vi "FlexMag - 23-03-2023.vi"() -> ()   [LabVIEW 2018] (continued)
                  n22734 = case shown="False" w26543 {
                    frame False {
                      n22735 = local read "process file list"() -> (w26547:string)
                      n22736 = Match Pattern(string=w26547, regular expression="1-)") -> (after substring=w26544:string)  [unwired: 1 in, 3 out]
                      n22737 = Equal?(x="", y=w26544) -> (x = y?=w26546:bool)
                      n22738 = case shown="False" w26546 {
                        frame False {
                          # "process done"
                          n22739 = flat-sequence {
                            frame #0 {
                              n22740 = local write "coating process done"(TRUE ("coating process done")) -> ()
                              n22741 = local write "Buzzer DO"(TRUE ("Buzzer DO")) -> ()
                              n22742 = local write "coating start"(FALSE ("coating start")) -> ()
                              n22743 = local write "Stop auto LN2"(TRUE ("Stop auto LN2")) -> ()
                              n22744 = local write "System Status"("DEPOSITION DONE" ("Warning Message")) -> ()
                              n22745 = Wait (ms)(milliseconds to wait=u32 3000) -> ()  [unwired: 1 out]
                            }
                            frame #1 {
                            }
                            frame #2 {
                              n22746 = Wait (ms)(milliseconds to wait=u32 1000) -> ()  [unwired: 1 out]
                              n22747 = local write "Buzzer DO"(FALSE ("Buzzer DO")) -> ()
                            }
                          }
                        }
                        frame True {
                          # "wrong file"
                          n22748 = flat-sequence {
                            frame #0 {
                              n22749 = local write "Buzzer DO"(TRUE ("Buzzer DO")) -> ()
                              n22750 = local write "coating process done"(TRUE ("coating process done")) -> ()
                              n22751 = Wait (ms)(milliseconds to wait=u32 3000) -> ()  [unwired: 1 out]
                              n22752 = local write "coating start"(FALSE ("coating start")) -> ()
                              n22753 = local write "Warning Message"("Please Enter a proper Process File !" ("Warning Message")) -> ()
                            }
                            frame #1 {
                            }
                            frame #2 {
                              n22754 = Wait (ms)(milliseconds to wait=u32 1000) -> ()  [unwired: 1 out]
                              n22755 = local write "Buzzer DO"(FALSE ("Buzzer DO")) -> ()
                            }
                          }
                        }
                      }
                    }
                    frame True {
                    }
                  }
                }
              }
            }
          }
        }
        n22756 = local write "coating process done"(FALSE ("coating process done")) -> ()
      }
    }
  }
  n22757 = while {
    stop <- FALSE stop-if-true
    n22758 = Wait Until Next ms Multiple(millisecond multiple=u32 300 ("milliseconds to wait")) -> ()  [unwired: 1 out]
    n22759 = case shown="True" "dcps check active" {
      frame False {
      }
      frame True {
        n22760 = local read "Dcps_is_on"() -> (w26575:bool)
        n22761 = feedback #343() -> (w26574:bool)  [unwired: 1 in]
        n22762 = case shown="True" w26575 {
          tunnel: w26574 -> [_ w26578]
          tunnel: [TRUE ("coating start") w26577] -> w26573
          frame False {
          }
          frame True {
            n22763 = local read "Actual DC Power : 2"() -> (w26580:dbl)
            n22764 = local read "Set DC Power auto"() -> (w26583:dbl)
            n22765 = Add(x="power difference", y=w26580) -> (x+y=w26585:dbl)
            n22766 = Subtract(x=w26580, y="power difference") -> (x-y=w26584:dbl)
            n22767 = In Range and Coerce(upper limit=w26585, x=w26583, lower limit=w26584) -> (In Range?=w26582:bool)  [unwired: 1 out]
            n22768 = Not(x=w26582) -> (.not. x?=w26581:bool)
            n22769 = case shown="True" w26581 {
              tunnel: w26578 -> [_ w26587]
              tunnel: [TRUE ("coating process done") FALSE ("coating start")] -> w26577
              frame False {
              }
              frame True {
                n22770 = call "Elapsed Time192"("Reset"=w26587) -> ("Elapsed Time (s)"=w26590:dbl)  [unwired: 11 in, 7 out]
                n22771 = Greater Or Equal?(x=w26590, y="dcps check(sec)") -> (x >= y?=w26589:bool)
                n22772 = case shown="True" w26589 {
                  frame False {
                  }
                  frame True {
                    n22773 = local read "coating start"() -> (w26594:bool)
                    n22774 = case shown="True" w26594 {
                      frame False {
                      }
                      frame True {
                        n22775 = local write "coating error"(TRUE ("coating error")) -> ()
                      }
                    }
                    n22776 = local write "Dc_auto_off"(TRUE ("Dc_auto_off")) -> ()
                    n22777 = local write "Warning Message"("No Actual  DC Power !" ("Warning Message")) -> ()
                  }
                }
              }
            }
          }
        }
        n22778 = feedback-in #343(w26573) -> ()
      }
    }
    n22779 = feedback #344() -> (w26568:bool)  [unwired: 1 in]
    n22780 = feedback #345() -> (w26569:bool)  [unwired: 1 in]
    n22781 = case shown="True" "coating error" {
      tunnel: [TRUE FALSE] -> w26567
      tunnel: w26568 -> [_ w26604]
      frame False {
      }
      frame True {
        n22782 = call "Elapsed Time156"("Auto Reset"=w26604) -> ("Elapsed Time (s)"=w26599:dbl)  [unwired: 11 in, 7 out]
        n22783 = In Range and Coerce(upper limit=7.0, x=w26599, lower limit=2.0) -> (In Range?=w26602:bool)  [unwired: 1 out]
        n22784 = In Range and Coerce(upper limit=1.5, x=w26599, lower limit=0.0) -> (In Range?=w26603:bool)  [unwired: 1 out]
        n22785 = In Range and Coerce(upper limit=10.0, x=w26599, lower limit=9.0) -> (In Range?=w26598:bool)  [unwired: 1 out]
        n22786 = case shown="True" w26603 {
          frame False {
          }
          frame True {
            w26622 = FALSE ("forward roll")
            w26623 = FALSE ("forward roll")
            n22787 = local write "coating process done"(TRUE ("coating process done")) -> ()
            n22788 = local write "Buzzer DO"(TRUE ("coating process done")) -> ()
            n22789 = local write "coating start"(FALSE ("coating start")) -> ()
            n22790 = local write "System Status"("COATING PROCESS CANCELLED !" ("System Status")) -> ()
            n22791 = local write "MFC_Ar_Set_value"(0.0 ("MFC_Ar_Set_value")) -> ()
            n22792 = local write "forward roll"(w26623) -> ()
            n22793 = local write "back roll"(w26623) -> ()
            n22794 = local write "CH1_Motor DO"(w26622) -> ()
            n22795 = local write "CH2_Motor DO"(w26622) -> ()
            n22796 = local write "CH3_Motor DO"(w26622) -> ()
            n22797 = local write "CH4_Motor DO"(w26622) -> ()
          }
        }
        n22798 = case shown="True" w26602 {
          frame False {
          }
          frame True {
            w26618 = TRUE ("Dc_auto_off")
            n22799 = local write "coating start"(FALSE ("coating start")) -> ()
            n22800 = local write "Dc_auto_off"(w26618) -> ()
            n22801 = local write "RF_auto_off"(w26618) -> ()
            n22802 = local write "MWPS1 auto close"(w26618) -> ()
            n22803 = local write "MWPS2 auto close"(w26618) -> ()
            n22804 = local write "MFC_Ar_Set"(TRUE ("MFC_Ar_Set")) -> ()
            n22805 = local write "Buzzer DO"(FALSE ("Buzzer DO")) -> ()
          }
        }
        n22806 = case shown="True" w26598 {
          frame False {
          }
          frame True {
            n22807 = local write "MFC_Ar_Set"(FALSE ("MFC_Ar_Set")) -> ()
            n22808 = local write "System Status"("SEMI-AUTOMATIC MODE" ("System Status")) -> ()
            n22809 = local write "coating error"(FALSE ("stop coating")) -> ()
          }
        }
        n22810 = local read "cassette position selection"() -> (w26597:u16)
        n22811 = case shown="4" w26597 {
          frame 0, Default {
          }
          frame 1 {
            n22812 = local write "pcgv1 auto open"(TRUE ("pcgv1 auto open")) -> ()
          }
          frame 2 {
            n22813 = local write "pcgv2 auto open"(TRUE ("pcgv2 auto open")) -> ()
          }
          frame 3 {
            n22814 = local write "pcgv3 auto open"(TRUE ("Dc_auto_off")) -> ()
          }
          frame 4 {
            n22815 = local write "pcgv4 auto open"(TRUE ("Dc_auto_off")) -> ()
          }
        }
      }
    }
    n22816 = feedback-in #344(w26567) -> ()
    n22817 = case shown="True" "stop coating" {
      tunnel: [TRUE FALSE] -> w26571
      tunnel: w26569 -> [_ w26636]
      frame False {
      }
      frame True {
        n22818 = call "Elapsed Time155"("Auto Reset"=w26636) -> ("Elapsed Time (s)"=w26631:dbl)  [unwired: 11 in, 7 out]
        n22819 = In Range and Coerce(upper limit=4.0, x=w26631, lower limit=2.0) -> (In Range?=w26634:bool)  [unwired: 1 out]
        n22820 = In Range and Coerce(upper limit=1.5, x=w26631, lower limit=0.0) -> (In Range?=w26635:bool)  [unwired: 1 out]
        n22821 = In Range and Coerce(upper limit=10.0, x=w26631, lower limit=7.0) -> (In Range?=w26630:bool)  [unwired: 1 out]
        n22822 = case shown="True" w26635 {
          frame False {
          }
          frame True {
            w26654 = FALSE ("forward roll")
            w26655 = FALSE ("forward roll")
            w26656 = TRUE ("coating process done")
            n22823 = local write "Buzzer DO"(w26656) -> ()
            n22824 = local write "coating process done"(w26656) -> ()
            n22825 = local write "coating start"(FALSE ("coating start")) -> ()
            n22826 = local write "System Status"("COATING PROCESS CANCELLED !" ("System Status")) -> ()
            n22827 = local write "MFC_Ar_Set_value"(0.0 ("MFC_Ar_Set_value")) -> ()
            n22828 = local write "forward roll"(w26655) -> ()
            n22829 = local write "back roll"(w26655) -> ()
            n22830 = local write "CH1_Motor DO"(w26654) -> ()
            n22831 = local write "CH2_Motor DO"(w26654) -> ()
            n22832 = local write "CH3_Motor DO"(w26654) -> ()
            n22833 = local write "CH4_Motor DO"(w26654) -> ()
          }
        }
        n22834 = case shown="True" w26634 {
          frame False {
          }
          frame True {
            w26650 = TRUE ("Dc_auto_off")
            n22835 = local write "coating start"(FALSE ("coating start")) -> ()
            n22836 = local write "Dc_auto_off"(w26650) -> ()
            n22837 = local write "RF_auto_off"(w26650) -> ()
            n22838 = local write "MWPS1 auto close"(w26650) -> ()
            n22839 = local write "MWPS2 auto close"(w26650) -> ()
            n22840 = local write "MFC_Ar_Set"(TRUE ("MFC_Ar_Set")) -> ()
            n22841 = local write "Buzzer DO"(FALSE ("Buzzer DO")) -> ()
          }
        }
        n22842 = case shown="True" w26630 {
          frame False {
          }
          frame True {
            n22843 = local write "MFC_Ar_Set"(FALSE ("MFC_Ar_Set")) -> ()
            n22844 = local write "stop coating"(FALSE ("stop coating")) -> ()
            n22845 = local write "System Status"("SEMI-AUTOMATIC MODE" ("System Status")) -> ()
          }
        }
        n22846 = local read "cassette position selection"() -> (w26629:u16)
        n22847 = case shown="4" w26629 {
          frame 0, Default {
          }
          frame 1 {
            n22848 = local write "pcgv1 auto open"(TRUE ("pcgv1 auto open")) -> ()
          }
          frame 2 {
            n22849 = local write "pcgv2 auto open"(TRUE ("pcgv2 auto open")) -> ()
          }
          frame 3 {
            n22850 = local write "pcgv3 auto open"(TRUE ("Dc_auto_off")) -> ()
          }
          frame 4 {
            n22851 = local write "pcgv4 auto open"(TRUE ("Dc_auto_off")) -> ()
          }
        }
      }
    }
    n22852 = feedback-in #345(w26571) -> ()
  }
  n22853 = while {
    stop <- FALSE stop-if-true
    n22854 = Wait Until Next ms Multiple(millisecond multiple=u32 300) -> ()  [unwired: 1 out]
    n22855 = case shown="True" "load process file" {
      frame False {
      }
      frame True {
        n22856 = stacked-sequence {
          seq-local: [w26670 _ _] -> [_ w26677 _]
          frame #0 {
            n22857 = call "File Dialog"("start path"=path "D:/VK-1701 System Files/Process Files") -> ("selected path"=w26672:path, "cancelled"=w26669:bool, "error out"=→"error out":errorcluster)  [unwired: 11 in, 1 out]
            n22858 = case shown="False" w26669 {
              tunnel: w26672 -> [w26675 _]
              tunnel: [w26674 string[][] [] ("all rows")] -> w26670
              frame False {
                n22859 = call-poly <vilib>:"Read Delimited Spreadsheet.vi"("file path (dialog if empty)"=w26675) -> ("all rows"=w26674:string[][])  [unwired: 9 in, 5 out]
              }
              frame True {
              }
            }
            "process counter" <- 0.0 ("Numeric")
            "process file list" <- "" ("process file list")
          }
          frame #1 {
            n22860 = while {
              tunnel: w26677 -> [w26683]
              i -> [w26682]
              stop <- w26679 stop-if-true
              n22861 = Index Array(array=w26683, index (row)=w26682, index (col)=0 ("disabled index (col)")) -> (element=w26678:string)
              n22862 = Equal?(x=w26678, y="") -> (x = y?=w26679:bool)
              n22863 = case shown="False" w26679 {
                tunnel: w26678 -> [w26684 _]
                frame False {
                  n22864 = local read "process file list"() -> (w26686:string)
                  n22865 = Concatenate Strings(w26686, "\r\n", w26684) -> (w26687:string)
                  n22866 = local write "process file list"(w26687) -> ()
                }
                frame True {
                }
              }
            }
          }
          frame #2 {
            n22867 = local read "process file list"() -> (w26690:string)
            n22868 = Match Pattern(string=w26690, regular expression="\r\n") -> (after substring=w26688:string)  [unwired: 1 in, 3 out]
            n22869 = local write "process file list"(w26688) -> ()
          }
        }
      }
    }
    n22870 = case shown="True" "creat recipe file" {
      frame False {
      }
      frame True {
        n22871 = call "FlexMag recipe file.vi"() -> ()  [unwired: 2 in]
      }
    }
    n22872 = case shown="True" "Change Rolling Direction" {
      frame False {
      }
      frame True {
        n22873 = local read "dep. for?"() -> (w26666:bool)
        n22874 = Not(x=w26666) -> (.not. x?=w26665:bool)
        n22875 = local write "dep. for?"(w26665) -> ()
        n22876 = local write "rolling direction gui"(w26665) -> ()
      }
    }
    n22877 = case shown="True" "creat process file" {
      frame False {
      }
      frame True {
        n22878 = call "FlexMag process file.vi"() -> ()  [unwired: 12 in]
      }
    }
  }
  n22879 = while {
    stop <- FALSE stop-if-true
    n22880 = Wait Until Next ms Multiple(millisecond multiple=u32 300) -> ()  [unwired: 1 out]
    n22881 = case shown="True" "CH1 LN2" {
      frame False {
      }
      frame True {
        n22882 = stacked-sequence {
          frame #0 {
            n22883 = local write "CH1_LN2_DO"(TRUE ("CH1_LN2_DO")) -> ()
            n22884 = Wait (ms)(milliseconds to wait=u32 100) -> ()  [unwired: 1 out]
          }
          frame #1 {
            n22885 = while {
              stop <- w26697 stop-if-true
              n22886 = stacked-sequence {
                frame #0 {
                  n22887 = while {
                    stop <- w26702 stop-if-true
                    n22888 = local read "ln2 ch1 top aim"() -> (w26704:dbl)
                    n22889 = local read "CH1_LN2_TK_t"() -> (w26705:u16)
                    n22890 = local read "CH1 LN2"() -> (w26703:bool)
                    n22891 = Greater Or Equal?(x=w26705, y=w26704) -> (x >= y?=w26701:bool)
                    n22892 = Not(x=w26703) -> (.not. x?=w26700:bool)
                    n22893 = Or(x=w26701, y=w26700) -> (x .or. y?=w26702:bool)
                    n22894 = Wait Until Next ms Multiple(millisecond multiple=u32 300) -> ()  [unwired: 1 out]
                  }
                }
                frame #1 {
                  n22895 = local write "CH1_LN2_DO"(FALSE ("CH1_LN2_DO")) -> ()
                  n22896 = Wait (ms)(milliseconds to wait=u32 100) -> ()  [unwired: 1 out]
                }
                frame #2 {
                  n22897 = while {
                    stop <- w26711 stop-if-true
                    n22898 = local read "ln2 ch1 bottom drop"() -> (w26713:dbl)
                    n22899 = local read "CH1_LN2_TK_b"() -> (w26714:u16)
                    n22900 = local read "CH1 LN2"() -> (w26712:bool)
                    n22901 = Less Or Equal?(x=w26714, y=w26713) -> (x <= y?=w26710:bool)
                    n22902 = Not(x=w26712) -> (.not. x?=w26709:bool)
                    n22903 = Or(x=w26710, y=w26709) -> (x .or. y?=w26711:bool)
                    n22904 = Wait Until Next ms Multiple(millisecond multiple=u32 300) -> ()  [unwired: 1 out]
                  }
                }
                frame #3 {
                  n22905 = local write "CH1_LN2_DO"(TRUE ("CH1_LN2_DO")) -> ()
                  n22906 = Wait (ms)(milliseconds to wait=u32 500) -> ()  [unwired: 1 out]
                }
                frame #4 {
                  n22907 = disable-structure shown="Disabled" {
                    frame Disabled {
                      n22908 = while {
                        stop <- w26721 stop-if-true
                        n22909 = local read "CH1_LN2_TK_t"() -> (w26723:u16)
                        n22910 = local read "ln2 dropdown"() -> (w26717:dbl)
                        n22911 = local read "CH1 LN2"() -> (w26722:bool)
                        n22912 = Less Or Equal?(x=w26723, y=w26717) -> (x <= y?=w26720:bool)
                        n22913 = Not(x=w26722) -> (.not. x?=w26719:bool)
                        n22914 = Or(x=w26720, y=w26719) -> (x .or. y?=w26721:bool)
                        n22915 = Wait Until Next ms Multiple(millisecond multiple=u32 300) -> ()  [unwired: 1 out]
                      }
                    }
                    frame Enabled {
                    }
                  }
                }
              }
              n22916 = Wait Until Next ms Multiple(millisecond multiple=u32 300) -> ()  [unwired: 1 out]
              n22917 = local read "CH1 LN2"() -> (w26698:bool)
              n22918 = Not(x=w26698) -> (.not. x?=w26697:bool)
            }
          }
          frame #2 {
            n22919 = local write "CH1_LN2_DO"(FALSE ("CH1_LN2_DO")) -> ()
            n22920 = Wait (ms)(milliseconds to wait=u32 100) -> ()  [unwired: 1 out]
          }
        }
      }
    }
  }
  n22921 = while {
    stop <- FALSE stop-if-true
    n22922 = Wait Until Next ms Multiple(millisecond multiple=u32 300) -> ()  [unwired: 1 out]
    n22923 = case shown="True" "CH2 LN2" {
      frame False {
      }
      frame True {
        n22924 = stacked-sequence {
          frame #0 {
            n22925 = local write "CH2_LN2_DO"(TRUE ("CH1_LN2_DO")) -> ()
            n22926 = Wait (ms)(milliseconds to wait=u32 100) -> ()  [unwired: 1 out]
          }
          frame #1 {
            n22927 = while {
              stop <- w26732 stop-if-true
              n22928 = stacked-sequence {
                frame #0 {
                  n22929 = while {
                    stop <- w26737 stop-if-true
                    n22930 = local read "ln2 ch2 top aim"() -> (w26739:dbl)
                    n22931 = local read "CH2_LN2_TK_t"() -> (w26740:u16)
                    n22932 = local read "CH2 LN2"() -> (w26738:bool)
                    n22933 = Greater Or Equal?(x=w26740, y=w26739) -> (x >= y?=w26736:bool)
                    n22934 = Not(x=w26738) -> (.not. x?=w26735:bool)
                    n22935 = Or(x=w26736, y=w26735) -> (x .or. y?=w26737:bool)
                    n22936 = Wait Until Next ms Multiple(millisecond multiple=u32 300) -> ()  [unwired: 1 out]
                  }
                }
                frame #1 {
                  n22937 = local write "CH2_LN2_DO"(FALSE ("CH1_LN2_DO")) -> ()
                  n22938 = Wait (ms)(milliseconds to wait=u32 100) -> ()  [unwired: 1 out]
                }
                frame #2 {
                  n22939 = while {
                    stop <- w26746 stop-if-true
                    n22940 = local read "ln2 ch3 bottom drop"() -> (w26748:dbl)
                    n22941 = local read "CH2_LN2_TK_b"() -> (w26749:u16)
                    n22942 = local read "CH2 LN2"() -> (w26747:bool)
                    n22943 = Less Or Equal?(x=w26749, y=w26748) -> (x <= y?=w26745:bool)
                    n22944 = Not(x=w26747) -> (.not. x?=w26744:bool)
                    n22945 = Or(x=w26745, y=w26744) -> (x .or. y?=w26746:bool)
                    n22946 = Wait Until Next ms Multiple(millisecond multiple=u32 300) -> ()  [unwired: 1 out]
                  }
                }
                frame #3 {
                  n22947 = local write "CH2_LN2_DO"(TRUE) -> ()
                  n22948 = Wait (ms)(milliseconds to wait=u32 500) -> ()  [unwired: 1 out]
                }
                frame #4 {
                  n22949 = disable-structure shown="Disabled" {
                    frame Disabled {
                      n22950 = while {
                        stop <- w26756 stop-if-true
                        n22951 = local read "CH2_LN2_TK_t"() -> (w26758:u16)
                        n22952 = local read "ln2 dropdown"() -> (w26752:dbl)
                        n22953 = local read "CH2 LN2"() -> (w26757:bool)
                        n22954 = Less Or Equal?(x=w26758, y=w26752) -> (x <= y?=w26755:bool)
                        n22955 = Not(x=w26757) -> (.not. x?=w26754:bool)
                        n22956 = Or(x=w26755, y=w26754) -> (x .or. y?=w26756:bool)
                        n22957 = Wait Until Next ms Multiple(millisecond multiple=u32 300) -> ()  [unwired: 1 out]
                      }
                    }
                    frame Enabled {
                    }
                  }
                }
              }
              n22958 = Wait Until Next ms Multiple(millisecond multiple=u32 300) -> ()  [unwired: 1 out]
              n22959 = local read "CH2 LN2"() -> (w26733:bool)
              n22960 = Not(x=w26733) -> (.not. x?=w26732:bool)
            }
          }
          frame #2 {
            n22961 = local write "CH2_LN2_DO"(FALSE ("CH2_LN2_DO")) -> ()
            n22962 = Wait (ms)(milliseconds to wait=u32 100) -> ()  [unwired: 1 out]
          }
        }
      }
    }
  }
  n22963 = while {
    stop <- FALSE stop-if-true
    n22964 = Wait Until Next ms Multiple(millisecond multiple=u32 300) -> ()  [unwired: 1 out]
    n22965 = case shown="True" "CH3 LN2" {
      frame False {
      }
      frame True {
        n22966 = stacked-sequence {
          frame #0 {
            n22967 = local write "CH3_LN2_DO"(TRUE ("CH1_LN2_DO")) -> ()
            n22968 = Wait (ms)(milliseconds to wait=u32 100) -> ()  [unwired: 1 out]
          }
          frame #1 {
            n22969 = while {
              stop <- w26767 stop-if-true
              n22970 = stacked-sequence {
                frame #0 {
                  n22971 = while {
                    stop <- w26772 stop-if-true
                    n22972 = local read "ln2 ch3 top aim"() -> (w26774:dbl)
                    n22973 = local read "CH3_LN2_TK_t"() -> (w26775:u16)
                    n22974 = local read "CH3 LN2"() -> (w26773:bool)
                    n22975 = Greater Or Equal?(x=w26775, y=w26774) -> (x >= y?=w26771:bool)
                    n22976 = Not(x=w26773) -> (.not. x?=w26770:bool)
                    n22977 = Or(x=w26771, y=w26770) -> (x .or. y?=w26772:bool)
                    n22978 = Wait Until Next ms Multiple(millisecond multiple=u32 300) -> ()  [unwired: 1 out]
                  }
                }
                frame #1 {
                  n22979 = local write "CH3_LN2_DO"(FALSE ("CH1_LN2_DO")) -> ()
                  n22980 = Wait (ms)(milliseconds to wait=u32 100) -> ()  [unwired: 1 out]
                }
                frame #2 {
                  n22981 = while {
                    stop <- w26781 stop-if-true
                    n22982 = local read "ln2 ch3 bottom drop"() -> (w26783:dbl)
                    n22983 = local read "CH3_LN2_TK_b"() -> (w26784:u16)
                    n22984 = local read "CH3 LN2"() -> (w26782:bool)
                    n22985 = Less Or Equal?(x=w26784, y=w26783) -> (x <= y?=w26780:bool)
                    n22986 = Not(x=w26782) -> (.not. x?=w26779:bool)
                    n22987 = Or(x=w26780, y=w26779) -> (x .or. y?=w26781:bool)
                    n22988 = Wait Until Next ms Multiple(millisecond multiple=u32 300) -> ()  [unwired: 1 out]
                  }
                }
                frame #3 {
                  n22989 = local write "CH3_LN2_DO"(TRUE) -> ()
                  n22990 = Wait (ms)(milliseconds to wait=u32 500) -> ()  [unwired: 1 out]
                }
                frame #4 {
                  n22991 = disable-structure shown="Disabled" {
                    frame Disabled {
                      n22992 = while {
                        stop <- w26791 stop-if-true
                        n22993 = local read "CH3_LN2_TK_t"() -> (w26793:u16)
                        n22994 = local read "ln2 dropdown"() -> (w26787:dbl)
                        n22995 = local read "CH3 LN2"() -> (w26792:bool)
                        n22996 = Less Or Equal?(x=w26793, y=w26787) -> (x <= y?=w26790:bool)
                        n22997 = Not(x=w26792) -> (.not. x?=w26789:bool)
                        n22998 = Or(x=w26790, y=w26789) -> (x .or. y?=w26791:bool)
                        n22999 = Wait Until Next ms Multiple(millisecond multiple=u32 300) -> ()  [unwired: 1 out]
                      }
                    }
                    frame Enabled {
                    }
                  }
                }
              }
              n23000 = Wait Until Next ms Multiple(millisecond multiple=u32 300) -> ()  [unwired: 1 out]
              n23001 = local read "CH3 LN2"() -> (w26768:bool)
              n23002 = Not(x=w26768) -> (.not. x?=w26767:bool)
            }
          }
          frame #2 {
            n23003 = local write "CH3_LN2_DO"(FALSE ("CH3_LN2_DO")) -> ()
            n23004 = Wait (ms)(milliseconds to wait=u32 100) -> ()  [unwired: 1 out]
          }
        }
      }
    }
  }
  n23005 = while {
    stop <- FALSE stop-if-true
    n23006 = Wait Until Next ms Multiple(millisecond multiple=u32 300) -> ()  [unwired: 1 out]
    n23007 = case shown="True" "CH4 LN2" {
      frame False {
      }
      frame True {
        n23008 = stacked-sequence {
          frame #0 {
            n23009 = local write "CH4_LN2_DO"(TRUE ("CH1_LN2_DO")) -> ()
            n23010 = Wait (ms)(milliseconds to wait=u32 100) -> ()  [unwired: 1 out]
          }
          frame #1 {
            n23011 = while {
              stop <- w26802 stop-if-true
              n23012 = stacked-sequence {
                frame #0 {
                  n23013 = while {
                    stop <- w26807 stop-if-true
                    n23014 = local read "ln2 ch4 top aim"() -> (w26809:dbl)
                    n23015 = local read "CH4_LN2_TK_t"() -> (w26810:u16)
                    n23016 = local read "CH4 LN2"() -> (w26808:bool)
                    n23017 = Greater Or Equal?(x=w26810, y=w26809) -> (x >= y?=w26806:bool)
                    n23018 = Not(x=w26808) -> (.not. x?=w26805:bool)
                    n23019 = Or(x=w26806, y=w26805) -> (x .or. y?=w26807:bool)
                    n23020 = Wait Until Next ms Multiple(millisecond multiple=u32 300) -> ()  [unwired: 1 out]
                  }
                }
                frame #1 {
                  n23021 = local write "CH4_LN2_DO"(FALSE ("CH1_LN2_DO")) -> ()
                  n23022 = Wait (ms)(milliseconds to wait=u32 100) -> ()  [unwired: 1 out]
                }
                frame #2 {
                  n23023 = while {
                    stop <- w26816 stop-if-true
                    n23024 = local read "ln2 ch4 bottom drop"() -> (w26818:dbl)
                    n23025 = local read "CH4_LN2_TK_b"() -> (w26819:u16)
                    n23026 = local read "CH4 LN2"() -> (w26817:bool)
                    n23027 = Less Or Equal?(x=w26819, y=w26818) -> (x <= y?=w26815:bool)
                    n23028 = Not(x=w26817) -> (.not. x?=w26814:bool)
                    n23029 = Or(x=w26815, y=w26814) -> (x .or. y?=w26816:bool)
                    n23030 = Wait Until Next ms Multiple(millisecond multiple=u32 300) -> ()  [unwired: 1 out]
                  }
                }
                frame #3 {
                  n23031 = local write "CH4_LN2_DO"(TRUE ("CH4_LN2_DO")) -> ()
                  n23032 = Wait (ms)(milliseconds to wait=u32 500) -> ()  [unwired: 1 out]
                }
                frame #4 {
                  n23033 = disable-structure shown="Disabled" {
                    frame Disabled {
                      n23034 = while {
                        stop <- w26826 stop-if-true
                        n23035 = local read "CH4_LN2_TK_t"() -> (w26828:u16)
                        n23036 = local read "ln2 dropdown"() -> (w26822:dbl)
                        n23037 = local read "CH4 LN2"() -> (w26827:bool)
                        n23038 = Less Or Equal?(x=w26828, y=w26822) -> (x <= y?=w26825:bool)
                        n23039 = Not(x=w26827) -> (.not. x?=w26824:bool)
                        n23040 = Or(x=w26825, y=w26824) -> (x .or. y?=w26826:bool)
                        n23041 = Wait Until Next ms Multiple(millisecond multiple=u32 300) -> ()  [unwired: 1 out]
                      }
                    }
                    frame Enabled {
                    }
                  }
                }
              }
              n23042 = Wait Until Next ms Multiple(millisecond multiple=u32 300) -> ()  [unwired: 1 out]
              n23043 = local read "CH4 LN2"() -> (w26803:bool)
              n23044 = Not(x=w26803) -> (.not. x?=w26802:bool)
            }
          }
          frame #2 {
            n23045 = local write "CH4_LN2_DO"(FALSE ("CH4_LN2_DO")) -> ()
            n23046 = Wait (ms)(milliseconds to wait=u32 100) -> ()  [unwired: 1 out]
          }
        }
      }
    }
  }
  n23047 = while {
    stop <- FALSE stop-if-true
    n23048 = Wait Until Next ms Multiple(millisecond multiple=u32 300) -> ()  [unwired: 1 out]
    n23049 = case shown="True" "Stop auto LN2" {
      frame False {
      }
      frame True {
        w26836 = FALSE ("CH1 LN2")
        w26837 = FALSE ("CH1 LN2")
        n23050 = local write "CH1_LN2_DO"(w26836) -> ()
        n23051 = local write "CH2_LN2_DO"(w26836) -> ()
        n23052 = local write "CH3_LN2_DO"(w26836) -> ()
        n23053 = local write "CH4_LN2_DO"(w26836) -> ()
        n23054 = local write "Stop auto LN2"(FALSE ("CH1 LN2")) -> ()
        n23055 = local write "CH1 LN2"(w26837) -> ()
        n23056 = local write "CH2 LN2"(w26837) -> ()
        n23057 = local write "CH3 LN2"(w26837) -> ()
        n23058 = local write "CH4 LN2"(w26837) -> ()
        n23059 = Wait (ms)(milliseconds to wait=u32 100) -> ()  [unwired: 1 out]
      }
    }
  }
  n23060 = while {
    stop <- FALSE stop-if-true
    n23061 = local read "CH1 LN2"() -> (w26842:bool)
    n23062 = local read "CH2 LN2"() -> (w26841:bool)
    n23063 = local read "CH3 LN2"() -> (w26840:bool)
    n23064 = local read "CH4 LN2"() -> (w26839:bool)
    n23065 = Wait Until Next ms Multiple(millisecond multiple=u32 1000) -> ()  [unwired: 1 out]
    n23066 = Compound Arithmetic op=OR(w26842, w26841, w26840, w26839) -> (w26843:bool)
    n23067 = case shown="True" w26843 {
      tunnel: [FALSE w26849] -> w26838
      frame False {
      }
      frame True {
        n23068 = local read "CH1_LN2_TK_b"() -> (w26863:u16)
        n23069 = local read "CH2_LN2_TK_b"() -> (w26856:u16)
        n23070 = local read "CH3_LN2_TK_b"() -> (w26858:u16)
        n23071 = local read "CH4_LN2_TK_b"() -> (w26859:u16)
        n23072 = local read "error level"() -> (w26862:dbl)
        n23073 = local read "error level"() -> (w26861:dbl)
        n23074 = local read "error level"() -> (w26857:dbl)
        n23075 = local read "error level"() -> (w26860:dbl)
        n23076 = Less Or Equal?(x=w26863, y=w26862) -> (x <= y?=w26855:bool)
        n23077 = Less Or Equal?(x=w26856, y=w26861) -> (x <= y?=w26853:bool)
        n23078 = Less Or Equal?(x=w26858, y=w26857) -> (x <= y?=w26852:bool)
        n23079 = Less Or Equal?(x=w26859, y=w26860) -> (x <= y?=w26851:bool)
        n23080 = Compound Arithmetic op=AND(w26855, w26853, w26852, w26851) -> (w26850:bool)
        n23081 = feedback #346() -> (w26864:bool)  [unwired: 1 in]
        n23082 = case shown="True" w26850 {
          tunnel: [TRUE FALSE] -> w26854
          tunnel: w26864 -> [_ w26870]
          tunnel: [FALSE w26871] -> w26849
          frame False {
          }
          frame True {
            n23083 = call "Elapsed Time189"("Reset"=w26870) -> ("Elapsed Time (s)"=w26872:dbl)  [unwired: 11 in, 7 out]
            n23084 = Multiply(x=60.0, y="dewar error time(min)") -> (x*y=w26869:dbl)
            n23085 = Greater Or Equal?(x=w26872, y=w26869) -> (x >= y?=w26871:bool)
          }
        }
        n23086 = feedback-in #346(w26854) -> ()
      }
    }
    n23087 = case shown="True" w26838 {
      frame False {
      }
      frame True {
        n23088 = local write "Warning Message"("Dewar is empty !") -> ()
        n23089 = local write "Stop auto LN2"(TRUE ("CH1 LN2")) -> ()
      }
    }
  }
  n23090 = VISA Close(VISA resource name=w60, error in (no error)=w61) -> ()  [unwired: 1 out]
  n23091 = while {
    stop <- FALSE stop-if-true
    n23092 = Wait Until Next ms Multiple(millisecond multiple=u32 300) -> ()  [unwired: 1 out]
    n23093 = case shown="True" "load recipe from path" {
      frame False {
      }
      frame True {
        n23094 = stacked-sequence {
          frame #0 {
            n23095 = local read "path for loading recipe"() -> (w27046:path)
            n23096 = call-poly <vilib>:"Read Delimited Spreadsheet.vi"("file path (dialog if empty)"=w27046) -> ("all rows"=w27166:string[][])  [unwired: 9 in, 5 out]
            n23097 = Index Array(array=w27166, index (row) #1=0 ("index (row)"), index (col) #1=4 ("index (row)"), index (row) #2=1 ("index (row)"), index (col) #2=4 ("index (row)"), index (row) #3=4 ("index (row)"), index (col) #3=4 ("index (row)"), index (row) #4=5 ("index (row)"), index (col) #4=4 ("index (row)"), index (row) #5=8 ("index (row)"), index (col) #5=4 ("index (row)"), index (row) #6=9 ("index (row)"), index (col) #6=4 ("index (row)"), index (row) #7=10 ("index (row)"), index (col) #7=4 ("index (row)"), index (row) #8=13 ("index (row)"), index (col) #8=4 ("index (row)"), index (row) #9=14 ("index (row)"), index (col) #9=4 ("index (row)"), index (row) #10=17 ("index (row)"), index (col) #10=4 ("index (row)"), index (row) #11=18 ("index (row)"), index (col) #11=4 ("index (row)"), index (row) #12=21 ("index (row)"), index (col) #12=4 ("index (row)"), index (row) #13=28 ("index (row)"), index (col) #13=4 ("index (row)"), index (row) #14=29 ("index (row)"), index (col) #14=4 ("index (row)"), index (row) #15=30 ("index (row)"), index (col) #15=4 ("index (row)"), index (row) #16=31 ("index (row)"), index (col) #16=4 ("index (row)"), index (row) #17=32 ("index (row)"), index (col) #17=4 ("index (row)"), index (row) #18=33 ("index (row)"), index (col) #18=4 ("index (row)"), index (row) #19=34 ("index (row)"), index (col) #19=4 ("index (row)"), index (row) #20=35 ("index (row)"), index (col) #20=4 ("index (row)"), index (row) #21=36 ("index (row)"), index (col) #21=4 ("index (row)"), index (row) #22=37 ("index (row)"), index (col) #22=4 ("index (row)"), index (row) #23=38 ("index (row)"), index (col) #23=4 ("index (row)"), index (row) #24=39 ("index (row)"), index (col) #24=4 ("index (row)"), index (row) #25=40 ("index (row)"), index (col) #25=4 ("index (row)"), index (row) #26=41 ("index (row)"), index (col) #26=4 ("index (row)"), index (row) #27=42 ("index (row)"), index (col) #27=4 ("index (row)"), index (row) #28=43 ("index (row)"), index (col) #28=4 ("index (row)"), index (row) #29=44 ("index (row)"), index (col) #29=4 ("index (row)"), index (row) #30=45 ("index (row)"), index (col) #30=4 ("index (row)"), index (row) #31=46 ("index (row)"), index (col) #31=4 ("index (row)"), index (row) #32=47 ("index (row)"), index (col) #32=4 ("index (row)"), index (row) #33=50 ("index (row)"), index (col) #33=4 ("index (row)"), index (row) #34=51 ("index (row)"), index (col) #34=4 ("index (row)"), index (row) #35=52 ("index (row)"), index (col) #35=4 ("index (row)"), index (row) #36=53 ("index (row)"), index (col) #36=4 ("index (row)"), index (row) #37=54 ("index (row)"), index (col) #37=4 ("index (row)"), index (row) #38=55 ("index (row)"), index (col) #38=4 ("index (row)"), index (row) #39=56 ("index (row)"), index (col) #39=4 ("index (row)"), index (row) #40=57 ("index (row)"), index (col) #40=4 ("index (row)"), index (row) #41=58 ("index (row)"), index (col) #41=4 ("index (row)"), index (row) #42=59 ("index (row)"), index (col) #42=4 ("index (row)"), index (row) #43=60 ("index (row)"), index (col) #43=4 ("index (row)"), index (row) #44=61 ("index (row)"), index (col) #44=4 ("index (row)"), index (row) #45=62 ("index (row)"), index (col) #45=4 ("index (row)"), index (row) #46=63 ("index (row)"), index (col) #46=4 ("index (row)"), index (row) #47=64 ("index (row)"), index (col) #47=4 ("index (row)"), index (row) #48=65 ("index (row)"), index (col) #48=4 ("index (row)"), index (row) #49=66 ("index (row)"), index (col) #49=4 ("index (row)"), index (row) #50=67 ("index (row)"), index (col) #50=4 ("index (row)"), index (row) #51=68 ("index (row)"), index (col) #51=4 ("index (row)"), index (row) #52=69 ("index (row)"), index (col) #52=4 ("index (row)"), index (row) #53=74 ("index (row)"), index (col) #53=4 ("index (row)"), index (row) #54=75 ("index (row)"), index (col) #54=4 ("index (row)"), index (row) #55=76 ("index (row)"), index (col) #55=4 ("index (row)"), index (row) #56=77 ("index (row)"), index (col) #56=4 ("index (row)"), index (row) #57=78 ("index (row)"), index (col) #57=4 ("index (row)"), index (row) #58=79 ("index (row)"), index (col) #58=4 ("index (row)"), index (row) #59=80 ("index (row)"), index (col) #59=4 ("index (row)"), index (row) #60=81 ("index (row)"), index (col) #60=4 ("index (row)"), index (row) #61=82 ("index (row)"), index (col) #61=4 ("index (row)"), index (row) #62=83 ("index (row)"), index (col) #62=4 ("index (row)"), index (row) #63=84 ("index (row)"), index (col) #63=4 ("index (row)"), index (row) #64=85 ("index (row)"), index (col) #64=4 ("index (row)"), index (row) #65=86 ("index (row)"), index (col) #65=4 ("index (row)"), index (row) #66=87 ("index (row)"), index (col) #66=4 ("index (row)"), index (row) #67=88 ("index (row)"), index (col) #67=4 ("index (row)"), index (row) #68=89 ("index (row)"), index (col) #68=4 ("index (row)"), index (row) #69=90 ("index (row)"), index (col) #69=4 ("index (row)"), index (row) #70=91 ("index (row)"), index (col) #70=4 ("index (row)"), index (row) #71=92 ("index (row)"), index (col) #71=4 ("index (row)"), index (row) #72=93 ("index (row)"), index (col) #72=4 ("index (row)"), index (row) #73=96 ("index (row)"), index (col) #73=4 ("index (row)"), index (row) #74=97 ("index (row)"), index (col) #74=4 ("index (row)"), index (row) #75=98 ("index (row)"), index (col) #75=4 ("index (row)"), index (row) #76=99 ("index (row)"), index (col) #76=4 ("index (row)"), index (row) #77=100 ("index (row)"), index (col) #77=4 ("index (row)"), index (row) #78=101 ("index (row)"), index (col) #78=4 ("index (row)"), index (row) #79=102 ("index (row)"), index (col) #79=4 ("index (row)"), index (row) #80=103 ("index (row)"), index (col) #80=4 ("index (row)"), index (row) #81=104 ("index (row)"), index (col) #81=4 ("index (row)"), index (row) #82=105 ("index (row)"), index (col) #82=4 ("index (row)"), index (row) #83=106 ("index (row)"), index (col) #83=4 ("index (row)"), index (row) #84=107 ("index (row)"), index (col) #84=4 ("index (row)"), index (row) #85=108 ("index (row)"), index (col) #85=4 ("index (row)"), index (row) #86=109 ("index (row)"), index (col) #86=4 ("index (row)"), index (row) #87=110 ("index (row)"), index (col) #87=4 ("index (row)"), index (row) #88=111 ("index (row)"), index (col) #88=4 ("index (row)"), index (row) #89=112 ("index (row)"), index (col) #89=4 ("index (row)"), index (row) #90=113 ("index (row)"), index (col) #90=4 ("index (row)"), index (row) #91=114 ("index (row)"), index (col) #91=4 ("index (row)"), index (row) #92=115 ("index (row)"), index (col) #92=4 ("index (row)"), index (row) #93=118 ("index (row)"), index (col) #93=4 ("index (row)"), index (row) #94=119 ("index (row)"), index (col) #94=4 ("index (row)"), index (row) #95=122 ("index (row)"), index (col) #95=4 ("index (row)"), index (row) #96=123 ("index (row)"), index (col) #96=4 ("index (row)")) -> (element #1=→"L recipe name":string, element #2=→"L sbs name":string, element #3=→"L recipe selection":string, element #4=→"L web selection":string, element #5=→"L core diamater":string, element #6=→"L left init diamater":string, element #7=→"L web thickness":string, element #8=→"L web speed":string, element #9=→"L tension  value":string, element #10=→"L single process type selection":string, element #11=→"L chamber selection":string, element #12=→"L microwave power":string, element #13=→"L dc power step 1":string, element #14=→"L dc power step 2":string, element #15=→"L dc power step 3":string, element #16=→"L dc power step 4":string, element #17=→"L dc power step 5":string, element #18=→"L dc power step 6":string, element #19=→"L dc power step 7":string, element #20=→"L dc power step 8":string, element #21=→"L dc power step 9":string, element #22=→"L dc power step 10":string, element #23=→"L dc power step 11":string, element #24=→"L dc power step 12":string, element #25=→"L dc power step 13":string, element #26=→"L dc power step 14":string, element #27=→"L dc power step 15":string, element #28=→"L dc power step 16":string, element #29=→"L dc power step 17":string, element #30=→"L dc power step 18":string, element #31=→"L dc power step 19":string, element #32=→"L dc power step 20":string, element #33=→"L dc length step 1":string, element #34=→"L dc length step 2":string, element #35=→"L dc length step 3":string, element #36=→"L dc length step 4":string, element #37=→"L dc length step 5":string, element #38=→"L dc length step 6":string, element #39=→"L dc length step 7":string, element #40=→"L dc length step 8":string, element #41=→"L dc length step 9":string, element #42=→"L dc length step 10":string, element #43=→"L dc length step 11":string, element #44=→"L dc length step 12":string, element #45=→"L dc length step 13":string, element #46=→"L dc length step 14":string, element #47=→"L dc length step 15":string, element #48=→"L dc length step 16":string, element #49=→"L dc length step 17":string, element #50=→"L dc length step 18":string, element #51=→"L dc length step 19":string, element #52=→"L dc length step 20":string, element #53=→"L rf power step 1":string, element #54=→"L rf power step 2":string, element #55=→"L rf power step 3":string, element #56=→"L rf power step 4":string, element #57=→"L rf power step 5":string, element #58=→"L rf power step 6":string, element #59=→"L rf power step 7":string, element #60=→"L rf power step 8":string, element #61=→"L rf power step 9":string, element #62=→"L rf power step 10":string, element #63=→"L rf power step 11":string, element #64=→"L rf power step 12":string, element #65=→"L rf power step 13":string, element #66=→"L rf power step 14":string, element #67=→"L rf power step 15":string, element #68=→"L rf power step 16":string, element #69=→"L rf power step 17":string, element #70=→"L rf power step 18":string, element #71=→"L rf power step 19":string, element #72=→"L rf power step 20":string, element #73=→"L rf length step 1":string, element #74=→"L rf length step 2":string, element #75=→"L rf length step 3":string, element #76=→"L rf length step 4":string, element #77=→"L rf length step 5":string, element #78=→"L rf length step 6":string, element #79=→"L rf length step 7":string, element #80=→"L rf length step 8":string, element #81=→"L rf length step 9":string, element #82=→"L rf length step 10":string, element #83=→"L rf length step 11":string, element #84=→"L rf length step 12":string, element #85=→"L rf length step 13":string, element #86=→"L rf length step 14":string, element #87=→"L rf length step 15":string, element #88=→"L rf length step 16":string, element #89=→"L rf length step 17":string, element #90=→"L rf length step 18":string, element #91=→"L rf length step 19":string, element #92=→"L rf length step 20":string, element #93=→"L argon flow":string, element #94=→"L pressure":string, element #95=→"L rf step numbers":string, element #96=→"L dc step numbers":string)
          }
          frame #1 {
            n23098 = local read "L single process type selection"() -> (w27184:string)
            n23099 = flat-sequence {
              frame #0 {
                n23100 = local read "L dc power step 20"() -> (w27264:string)
                n23101 = local read "L dc power step 19"() -> (w27257:string)
                n23102 = local read "L dc power step 18"() -> (w27258:string)
                n23103 = local read "L dc power step 11"() -> (w27250:string)
                n23104 = local read "L dc power step 17"() -> (w27262:string)
                n23105 = local read "L dc power step 12"() -> (w27249:string)
                n23106 = local read "L dc power step 14"() -> (w27254:string)
                n23107 = local read "L dc power step 10"() -> (w27352:string)
                n23108 = local read "L dc power step 13"() -> (w27253:string)
                n23109 = local read "L dc power step 15"() -> (w27267:string)
                n23110 = local read "L dc power step 16"() -> (w27261:string)
                n23111 = local read "L dc power step 9"() -> (w27359:string)
                n23112 = local read "L dc power step 8"() -> (w27358:string)
                n23113 = local read "L dc power step 1"() -> (w27366:string)
                n23114 = local read "L dc power step 7"() -> (w27354:string)
                n23115 = local read "L dc power step 2"() -> (w27367:string)
                n23116 = local read "L dc power step 4"() -> (w27362:string)
                n23117 = local read "L dc power step 3"() -> (w27363:string)
                n23118 = local read "L dc power step 5"() -> (w27349:string)
                n23119 = local read "L dc power step 6"() -> (w27355:string)
                n23120 = Wait (ms)(milliseconds to wait=u32 1000) -> ()  [unwired: 1 out]
                n23121 = Decimal String To Number(string=w27264) -> (number=w27265:i32)  [unwired: 2 in, 1 out]
                n23122 = Decimal String To Number(string=w27257) -> (number=w27256:i32)  [unwired: 2 in, 1 out]
                n23123 = Decimal String To Number(string=w27258) -> (number=w27259:i32)  [unwired: 2 in, 1 out]
                n23124 = Decimal String To Number(string=w27250) -> (number=w27251:i32)  [unwired: 2 in, 1 out]
                n23125 = Decimal String To Number(string=w27262) -> (number=w27263:i32)  [unwired: 2 in, 1 out]
                n23126 = Decimal String To Number(string=w27249) -> (number=w27248:i32)  [unwired: 2 in, 1 out]
                n23127 = Decimal String To Number(string=w27254) -> (number=w27255:i32)  [unwired: 2 in, 1 out]
                n23128 = Decimal String To Number(string=w27352) -> (number=w27351:i32)  [unwired: 2 in, 1 out]
                n23129 = Decimal String To Number(string=w27253) -> (number=w27252:i32)  [unwired: 2 in, 1 out]
                n23130 = Decimal String To Number(string=w27267) -> (number=w27266:i32)  [unwired: 2 in, 1 out]
                n23131 = Decimal String To Number(string=w27261) -> (number=w27260:i32)  [unwired: 2 in, 1 out]
                n23132 = Decimal String To Number(string=w27359) -> (number=w27360:i32)  [unwired: 2 in, 1 out]
                n23133 = Decimal String To Number(string=w27358) -> (number=w27357:i32)  [unwired: 2 in, 1 out]
                n23134 = Decimal String To Number(string=w27366) -> (number=w27365:i32)  [unwired: 2 in, 1 out]
                n23135 = Decimal String To Number(string=w27354) -> (number=w27353:i32)  [unwired: 2 in, 1 out]
                n23136 = Decimal String To Number(string=w27367) -> (number=w27368:i32)  [unwired: 2 in, 1 out]
                n23137 = Decimal String To Number(string=w27362) -> (number=w27361:i32)  [unwired: 2 in, 1 out]
                n23138 = Decimal String To Number(string=w27363) -> (number=w27364:i32)  [unwired: 2 in, 1 out]
                n23139 = Decimal String To Number(string=w27349) -> (number=w27350:i32)  [unwired: 2 in, 1 out]
                n23140 = Decimal String To Number(string=w27355) -> (number=w27356:i32)  [unwired: 2 in, 1 out]
                n23141 = local write "R dc step power 20"(w27265) -> ()
                n23142 = local write "R dc step power 19"(w27256) -> ()
                n23143 = local write "R dc step power 18"(w27259) -> ()
                n23144 = local write "R dc step power 11"(w27251) -> ()
                n23145 = local write "R dc step power 17"(w27263) -> ()
                n23146 = local write "R dc step power 12"(w27248) -> ()
                n23147 = local write "R dc step power 14"(w27255) -> ()
                n23148 = local write "R dc step power 10"(w27351) -> ()
                n23149 = local write "R dc step power 13"(w27252) -> ()
                n23150 = local write "R dc step power 15"(w27266) -> ()
                n23151 = local write "R dc step power 16"(w27260) -> ()
                n23152 = local write "R dc step power 9"(w27360) -> ()
                n23153 = local write "R dc step power 1"(w27365) -> ()
                n23154 = local write "R dc step power 8"(w27357) -> ()
                n23155 = local write "R dc step power 7"(w27353) -> ()
                n23156 = local write "R dc step power 2"(w27368) -> ()
                n23157 = local write "R dc step power 4"(w27361) -> ()
                n23158 = local write "R dc step power 3"(w27364) -> ()
                n23159 = local write "R dc step power 5"(w27350) -> ()
                n23160 = local write "R dc step power 6"(w27356) -> ()
                n23161 = local read "L dc length step 11"() -> (w27285:string)
                n23162 = local read "L dc length step 17"() -> (w27273:string)
                n23163 = local read "L dc length step 12"() -> (w27286:string)
                n23164 = local read "L dc length step 14"() -> (w27281:string)
                n23165 = local read "L dc length step 19"() -> (w27278:string)
                n23166 = local read "L dc length step 20"() -> (w27271:string)
                n23167 = local read "L dc length step 13"() -> (w27282:string)
                n23168 = local read "L dc length step 15"() -> (w27268:string)
                n23169 = local read "L dc length step 16"() -> (w27274:string)
                n23170 = local read "L dc length step 18"() -> (w27277:string)
                n23171 = local read "L dc length step 1"() -> (w27331:string)
                n23172 = local read "L dc length step 10"() -> (w27345:string)
                n23173 = local read "L dc length step 7"() -> (w27343:string)
                n23174 = local read "L dc length step 2"() -> (w27330:string)
                n23175 = local read "L dc length step 4"() -> (w27335:string)
                n23176 = local read "L dc length step 9"() -> (w27338:string)
                n23177 = local read "L dc length step 3"() -> (w27334:string)
                n23178 = local read "L dc length step 5"() -> (w27348:string)
                n23179 = local read "L dc length step 6"() -> (w27342:string)
                n23180 = local read "L dc length step 8"() -> (w27339:string)
                n23181 = Decimal String To Number(string=w27285) -> (number=w27284:i32)  [unwired: 2 in, 1 out]
                n23182 = Decimal String To Number(string=w27273) -> (number=w27272:i32)  [unwired: 2 in, 1 out]
                n23183 = Decimal String To Number(string=w27286) -> (number=w27287:i32)  [unwired: 2 in, 1 out]
                n23184 = Decimal String To Number(string=w27281) -> (number=w27280:i32)  [unwired: 2 in, 1 out]
                n23185 = Decimal String To Number(string=w27278) -> (number=w27279:i32)  [unwired: 2 in, 1 out]
                n23186 = Decimal String To Number(string=w27271) -> (number=w27270:i32)  [unwired: 2 in, 1 out]
                n23187 = Decimal String To Number(string=w27282) -> (number=w27283:i32)  [unwired: 2 in, 1 out]
                n23188 = Decimal String To Number(string=w27268) -> (number=w27269:i32)  [unwired: 2 in, 1 out]
                n23189 = Decimal String To Number(string=w27274) -> (number=w27275:i32)  [unwired: 2 in, 1 out]
                n23190 = Decimal String To Number(string=w27277) -> (number=w27276:i32)  [unwired: 2 in, 1 out]
                n23191 = Decimal String To Number(string=w27331) -> (number=w27332:i32)  [unwired: 2 in, 1 out]
                n23192 = Decimal String To Number(string=w27343) -> (number=w27344:i32)  [unwired: 2 in, 1 out]
                n23193 = Decimal String To Number(string=w27330) -> (number=w27329:i32)  [unwired: 2 in, 1 out]
                n23194 = Decimal String To Number(string=w27335) -> (number=w27336:i32)  [unwired: 2 in, 1 out]
                n23195 = Decimal String To Number(string=w27338) -> (number=w27337:i32)  [unwired: 2 in, 1 out]
                n23196 = Decimal String To Number(string=w27345) -> (number=w27346:i32)  [unwired: 2 in, 1 out]
                n23197 = Decimal String To Number(string=w27334) -> (number=w27333:i32)  [unwired: 2 in, 1 out]
                n23198 = Decimal String To Number(string=w27348) -> (number=w27347:i32)  [unwired: 2 in, 1 out]
                n23199 = Decimal String To Number(string=w27342) -> (number=w27341:i32)  [unwired: 2 in, 1 out]
                n23200 = Decimal String To Number(string=w27339) -> (number=w27340:i32)  [unwired: 2 in, 1 out]
                n23201 = local write "R dc step length 11"(w27284) -> ()
                n23202 = local write "R dc step length 17"(w27272) -> ()
                n23203 = local write "R dc step length 12"(w27287) -> ()
                n23204 = local write "R dc step length 14"(w27280) -> ()
                n23205 = local write "R dc step length 19"(w27279) -> ()
                n23206 = local write "R dc step length 20"(w27270) -> ()
                n23207 = local write "R dc step length 13"(w27283) -> ()
                n23208 = local write "R dc step length 15"(w27269) -> ()
                n23209 = local write "R dc step length 16"(w27275) -> ()
                n23210 = local write "R dc step length 18"(w27276) -> ()
                n23211 = local write "R dc step length 1"(w27332) -> ()
                n23212 = local write "R dc step length 10"(w27346) -> ()
                n23213 = local write "R dc step length 7"(w27344) -> ()
                n23214 = local write "R dc step length 2"(w27329) -> ()
                n23215 = local write "R dc step length 4"(w27336) -> ()
                n23216 = local write "R dc step length 9"(w27337) -> ()
                n23217 = local write "R dc step length 3"(w27333) -> ()
                n23218 = local write "R dc step length 5"(w27347) -> ()
                n23219 = local write "R dc step length 6"(w27341) -> ()
                n23220 = local write "R dc step length 8"(w27340) -> ()
                n23221 = local read "L rf power step 10"() -> (w27231:string)
                n23222 = local read "L rf power step 10"() -> (w27304:string)
                n23223 = local read "L rf power step 9"() -> (w27238:string)
                n23224 = local read "L rf power step 9"() -> (w27297:string)
                n23225 = local read "L rf power step 8"() -> (w27237:string)
                n23226 = local read "L rf power step 8"() -> (w27298:string)
                n23227 = local read "L rf power step 1"() -> (w27245:string)
                n23228 = local read "L rf power step 7"() -> (w27233:string)